vi "SaccadeAnalyser - Main.vi"(8 "error in (no error)":errorcluster, 11 "Data IN":T3={"Impulse Positions"=[{"Start"=5471, "End"=5813, "Impulse Plane"=enum."Yaw", "Impulse Direction +ve?"=FALSE, "Time offset"=0, "Amplitude offset"=0.0}, {"Start"=6974, "End"=7325, "Impulse Plane"=enum."Yaw", "Impulse Direction +ve?"=TRUE, "Time offset"=0, "Amplitude offset"=0.0}, {"Start"=7641, "End"=7980, "Impulse Plane"=enum."Yaw", "Impulse Direction +ve?"=FALSE, "Time offset"=0, "Amplitude offset"=0.0}, {"Start"=9060, "End"=9400, "Impulse Plane"=enum."Yaw", "Impulse Direction +ve?"=FALSE, "Time offset"=0, "Amplitude offset"=0.0}, {"Start"=9938, "End"=10282, "Impulse Plane"=enum."Yaw", "Impulse Direction +ve?"=FALSE, "Time offset"=0, "Amplitude offset"=0.0}, {"Start"=10800, "End"=11142, "Impulse Plane"=enum."Yaw", "Impulse Direction +ve?"=FALSE, "Time offset"=0, "Amplitude offset"=0.0}, {"Start"=11602, "End"=11942, "Impulse Plane"=enum."Yaw", "Impulse Direction +ve?"=TRUE, "Time offset"=0, "Amplitude offset"=0.0}, {"Start"=12449, "End"=12790, "Impulse Plane"=enum."Yaw", "Impulse Direction +ve?"=TRUE, "Time offset"=0, "Amplitude offset"=0.0}, {"Start"=13310, "End"=13653, "Impulse Plane"=enum."Yaw", "Impulse Direction +ve?"=TRUE, "Time offset"=0, "Amplitude offset"=0.0}, {"Start"=14191, "End"=14535, "Impulse Plane"=enum."Yaw", "Impulse Direction +ve?"=TRUE, "Time offset"=0, "Amplitude offset"=0.0}, {"Start"=15040, "End"=15380, "Impulse Plane"=enum."Yaw", "Impulse Direction +ve?"=FALSE, "Time offset"=0, "Amplitude offset"=0.0}, {"Start"=16780, "End"=17124, "Impulse Plane"=enum."Yaw", "Impulse Direction +ve?"=TRUE, "Time offset"=0, "Amplitude offset"=0.0}, {"Start"=17572, "End"=17913, "Impulse Plane"=enum."Yaw", "Impulse Direction +ve?"=FALSE, "Time offset"=0, "Amplitude offset"=0.0}, {"Start"=18369, "End"=18713, "Impulse Plane"=enum."Yaw", "Impulse Direction +ve?"=FALSE, "Time offset"=0, "Amplitude offset"=0.0}, {"Start"=19174, "End"=19519, "Impulse Plane"=enum."Yaw", "Impulse Direction +ve?"=FALSE, "Time offset"=0, "Amplitude offset"=0.0}, {"Start"=19928, "End"=20270, "Impulse Plane"=enum."Yaw", "Impulse Direction +ve?"=TRUE, "Time offset"=0, "Amplitude offset"=0.0}, {"Start"=20762, "End"=21121, "Impulse Plane"=enum."Yaw", "Impulse Direction +ve?"=FALSE, "Time offset"=0, "Amplitude offset"=0.0}, {"Start"=21554, "End"=21888, "Impulse Plane"=enum."Yaw", "Impulse Direction +ve?"=FALSE, "Time offset"=0, "Amplitude offset"=0.0}, {"Start"=22293, "End"=22639, "Impulse Plane"=enum."Yaw", "Impulse Direction +ve?"=TRUE, "Time offset"=0, "Amplitude offset"=0.0}, {"Start"=23109, "End"=23464, "Impulse Plane"=enum."Yaw", "Impulse Direction +ve?"=TRUE, "Time offset"=0, "Amplitude offset"=0.0}, {"Start"=23868, "End"=24215, "Impulse Plane"=enum."Yaw", "Impulse Direction +ve?"=TRUE, "Time offset"=0, "Amplitude offset"=0.0}, {"Start"=24643, "End"=24992, "Impulse Plane"=enum."Yaw", "Impulse Direction +ve?"=FALSE, "Time offset"=0, "Amplitude offset"=0.0}, {"Start"=25685, "End"=26023, "Impulse Plane"=enum."Yaw", "Impulse Direction +ve?"=FALSE, "Time offset"=0, "Amplitude offset"=0.0}, {"Start"=26431, "End"=26768, "Impulse Plane"=enum."Yaw", "Impulse Direction +ve?"=FALSE, "Time offset"=0, "Amplitude offset"=0.0}, {"Start"=27251, "End"=27595, "Impulse Plane"=enum."Yaw", "Impulse Direction +ve?"=FALSE, "Time offset"=0, "Amplitude offset"=0.0}, {"Start"=28832, "End"=29180, "Impulse Plane"=enum."Yaw", "Impulse Direction +ve?"=TRUE, "Time offset"=0, "Amplitude offset"=0.0}, {"Start"=31028, "End"=31383, "Impulse Plane"=enum."LARP", "Impulse Direction +ve?"=FALSE, "Time offset"=0, "Amplitude offset"=0.0}, {"Start"=32603, "End"=32936, "Impulse Plane"=enum."LARP", "Impulse Direction +ve?"=TRUE, "Time offset"=0, "Amplitude offset"=0.0}, {"Start"=33445, "End"=33779, "Impulse Plane"=enum."LARP", "Impulse Direction +ve?"=TRUE, "Time offset"=0, "Amplitude offset"=0.0}, {"Start"=34276, "End"=34629, "Impulse Plane"=enum."LARP", "Impulse Direction +ve?"=FALSE, "Time offset"=0, "Amplitude offset"=0.0}, {"Start"=35114, "End"=35460, "Impulse Plane"=enum."LARP", "Impulse Direction +ve?"=FALSE, "Time offset"=0, "Amplitude offset"=0.0}, {"Start"=35981, "End"=36324, "Impulse Plane"=enum."LARP", "Impulse Direction +ve?"=TRUE, "Time offset"=0, "Amplitude offset"=0.0}, {"Start"=36920, "End"=37249, "Impulse Plane"=enum."LARP", "Impulse Direction +ve?"=TRUE, "Time offset"=0, "Amplitude offset"=0.0}, {"Start"=37988, "End"=38322, "Impulse Plane"=enum."LARP", "Impulse Direction +ve?"=TRUE, "Time offset"=0, "Amplitude offset"=0.0}, {"Start"=38964, "End"=39324, "Impulse Plane"=enum."LARP", "Impulse Direction +ve?"=FALSE, "Time offset"=0, "Amplitude offset"=0.0}, {"Start"=39948, "End"=40284, "Impulse Plane"=enum."LARP", "Impulse Direction +ve?"=TRUE, "Time offset"=0, "Amplitude offset"=0.0}, {"Start"=40958, "End"=41293, "Impulse Plane"=enum."LARP", "Impulse Direction +ve?"=TRUE, "Time offset"=0, "Amplitude offset"=0.0}, {"Start"=41899, "End"=42229, "Impulse Plane"=enum."LARP", "Impulse Direction +ve?"=TRUE, "Time offset"=0, "Amplitude offset"=0.0}, {"Start"=42801, "End"=43154, "Impulse Plane"=enum."LARP", "Impulse Direction +ve?"=FALSE, "Time offset"=0, "Amplitude offset"=0.0}, {"Start"=43641, "End"=43980, "Impulse Plane"=enum."LARP", "Impulse Direction +ve?"=TRUE, "Time offset"=0, "Amplitude offset"=0.0}, {"Start"=44466, "End"=44821, "Impulse Plane"=enum."LARP", "Impulse Direction +ve?"=FALSE, "Time offset"=0, "Amplitude offset"=0.0}, {"Start"=45388, "End"=45722, "Impulse Plane"=enum."LARP", "Impulse Direction +ve?"=TRUE, "Time offset"=0, "Amplitude offset"=0.0}, {"Start"=46149, "End"=46510, "Impulse Plane"=enum."LARP", "Impulse Direction +ve?"=FALSE, "Time offset"=0, "Amplitude offset"=0.0}, {"Start"=47874, "End"=48206, "Impulse Plane"=enum."LARP", "Impulse Direction +ve?"=TRUE, "Time offset"=0, "Amplitude offset"=0.0}, {"Start"=50143, "End"=50479, "Impulse Plane"=enum."RALP", "Impulse Direction +ve?"=TRUE, "Time offset"=0, "Amplitude offset"=0.0}, {"Start"=50976, "End"=51310, "Impulse Plane"=enum."RALP", "Impulse Direction +ve?"=FALSE, "Time offset"=0, "Amplitude offset"=0.0}, {"Start"=51892, "End"=52226, "Impulse Plane"=enum."RALP", "Impulse Direction +ve?"=FALSE, "Time offset"=0, "Amplitude offset"=0.0}, {"Start"=52839, "End"=53171, "Impulse Plane"=enum."RALP", "Impulse Direction +ve?"=FALSE, "Time offset"=0, "Amplitude offset"=0.0}, {"Start"=53676, "End"=54012, "Impulse Plane"=enum."RALP", "Impulse Direction +ve?"=TRUE, "Time offset"=0, "Amplitude offset"=0.0}, {"Start"=54530, "End"=54877, "Impulse Plane"=enum."RALP", "Impulse Direction +ve?"=FALSE, "Time offset"=0, "Amplitude offset"=0.0}, {"Start"=55371, "End"=55711, "Impulse Plane"=enum."RALP", "Impulse Direction +ve?"=TRUE, "Time offset"=0, "Amplitude offset"=0.0}, {"Start"=56153, "End"=56482, "Impulse Plane"=enum."RALP", "Impulse Direction +ve?"=FALSE, "Time offset"=0, "Amplitude offset"=0.0}, {"Start"=57053, "End"=57390, "Impulse Plane"=enum."RALP", "Impulse Direction +ve?"=FALSE, "Time offset"=0, "Amplitude offset"=0.0}, {"Start"=57954, "End"=58292, "Impulse Plane"=enum."RALP", "Impulse Direction +ve?"=FALSE, "Time offset"=0, "Amplitude offset"=0.0}, {"Start"=58794, "End"=59130, "Impulse Plane"=enum."RALP", "Impulse Direction +ve?"=TRUE, "Time offset"=0, "Amplitude offset"=0.0}, {"Start"=59587, "End"=59931, "Impulse Plane"=enum."RALP", "Impulse Direction +ve?"=TRUE, "Time offset"=0, "Amplitude offset"=0.0}, {"Start"=60399, "End"=60744, "Impulse Plane"=enum."RALP", "Impulse Direction +ve?"=FALSE, "Time offset"=0, "Amplitude offset"=0.0}, {"Start"=61218, "End"=61559, "Impulse Plane"=enum."RALP", "Impulse Direction +ve?"=FALSE, "Time offset"=0, "Amplitude offset"=0.0}, {"Start"=62100, "End"=62442, "Impulse Plane"=enum."RALP", "Impulse Direction +ve?"=FALSE, "Time offset"=0, "Amplitude offset"=0.0}, {"Start"=62989, "End"=63322, "Impulse Plane"=enum."RALP", "Impulse Direction +ve?"=FALSE, "Time offset"=0, "Amplitude offset"=0.0}, {"Start"=63787, "End"=64136, "Impulse Plane"=enum."RALP", "Impulse Direction +ve?"=TRUE, "Time offset"=0, "Amplitude offset"=0.0}, {"Start"=64603, "End"=64953, "Impulse Plane"=enum."RALP", "Impulse Direction +ve?"=FALSE, "Time offset"=0, "Amplitude offset"=0.0}, {"Start"=65462, "End"=65795, "Impulse Plane"=enum."RALP", "Impulse Direction +ve?"=FALSE, "Time offset"=0, "Amplitude offset"=0.0}, {"Start"=66308, "End"=66645, "Impulse Plane"=enum."RALP", "Impulse Direction +ve?"=FALSE, "Time offset"=0, "Amplitude offset"=0.0}, {"Start"=67052, "End"=67402, "Impulse Plane"=enum."RALP", "Impulse Direction +ve?"=TRUE, "Time offset"=0, "Amplitude offset"=0.0}], "No. Imp"=15, "Parameter Time Series"=[{"time offset"=0.0, "Offset"=0.0, "Gain"=1.0, "inverse"=FALSE, "filter data"=FALSE, "dots"=FALSE, "interpolate"=FALSE, "List 1"=5, "Color Box"=6618880, "Boolean"=TRUE}, {"time offset"=0.0, "Offset"=0.0, "Gain"=1.0, "inverse"=FALSE, "filter data"=FALSE, "dots"=FALSE, "interpolate"=FALSE, "List 1"=6, "Color Box"=6618880, "Boolean"=FALSE}, {"time offset"=0.0, "Offset"=0.0, "Gain"=1.0, "inverse"=FALSE, "filter data"=FALSE, "dots"=FALSE, "interpolate"=FALSE, "List 1"=7, "Color Box"=6618880, "Boolean"=FALSE}, {"time offset"=0.0, "Offset"=0.0, "Gain"=1.0, "inverse"=FALSE, "filter data"=FALSE, "dots"=FALSE, "interpolate"=FALSE, "List 1"=13, "Color Box"=16777224, "Boolean"=TRUE}, {"time offset"=0.0, "Offset"=0.0, "Gain"=1.0, "inverse"=FALSE, "filter data"=FALSE, "dots"=FALSE, "interpolate"=FALSE, "List 1"=14, "Color Box"=16777224, "Boolean"=FALSE}, {"time offset"=0.0, "Offset"=0.0, "Gain"=1.0, "inverse"=FALSE, "filter data"=FALSE, "dots"=FALSE, "interpolate"=FALSE, "List 1"=15, "Color Box"=16777224, "Boolean"=FALSE}], "Parameter Impuls Series"=[{"Color"=6618880, "Visible"=TRUE, "Channel"=1, "Invert"=FALSE, "Desaccade"=FALSE, "Offset"=0.0, "Gain"=1.0}, {"Color"=6618880, "Visible"=FALSE, "Channel"=6, "Invert"=FALSE, "Desaccade"=FALSE, "Offset"=0.0, "Gain"=1.0}, {"Color"=6618880, "Visible"=FALSE, "Channel"=7, "Invert"=FALSE, "Desaccade"=FALSE, "Offset"=0.0, "Gain"=1.0}, {"Color"=16777224, "Visible"=TRUE, "Channel"=13, "Invert"=FALSE, "Desaccade"=FALSE, "Offset"=0.0, "Gain"=1.0}, {"Color"=16777224, "Visible"=FALSE, "Channel"=14, "Invert"=FALSE, "Desaccade"=FALSE, "Offset"=0.0, "Gain"=1.0}, {"Color"=16777224, "Visible"=FALSE, "Channel"=15, "Invert"=FALSE, "Desaccade"=FALSE, "Offset"=0.0, "Gain"=1.0}], "Experiment Parameters"={"Freq"=0.0, "Vel"=0, "Acc"=0, "Stimulus"="Head Impulse"}, "Autosort File"=refnum, "Data File"={"Data Channels"=array34x71049[2415666 elements], "Sample Rate"=500, "Channel List"=["Hz Position-in-Head", "Hz Velocity-in-Head", "Hy Position-in-Head", "Hy Velocity-in-Head", "Hx Position-in-Head", "Hx Velocity-in-Head", "Hl Velocity-in-Head", "Hr Velocity-in-Head", "Lx Position-in-Head", "Ly Position-in-Head", "Lz Position-in-Head", "Lx Velocity-in-Head", "Ly Velocity-in-Head", "Lz Velocity-in-Head", "Ll Velocity-in-Head", "Lr Velocity-in-Head", "Rx Position-in-Head", "Ry Position-in-Head", "Rz Position-in-Head", "Rx Velocity-in-Head", "Ry Velocity-in-Head", "Rz Velocity-in-Head", "Rl Velocity-in-Head", "Rr Velocity-in-Head", "Target on/off", "aux input 1", "aux input 2", " ", "", "", "", "Target Hor", "Target Ver", ""]}, "Experiment data path"=path "C:/Users/w.figtree/Desktop/Coils Data/3", "Image data path"=path "/Macintosh HD/Users/patrick/Studium/Diploma Thesis/Data Analysis", "LVS data path"=path "/Macintosh HD/Users/patrick/Studium/Diploma Thesis/Data Analysis", "Raw copy path"=path "/Macintosh HD/Users/patrick/Studium/Diploma Thesis/Data Analysis", "filename"="passive_lvs.lvs", "desaccading parameters"={"Tolerance"=3, "Acc Range"=7000.0, "Sample Rate"=500, "Impulse Plane 2"=enum."Yaw", "Impulse dir"=FALSE}, "Experiment Parameters 2"={"Subject"="SE Trial Short Term", "Strain"="", "Rotation plane"="", "Experimenter"=" ", "Trial"=0.0, "Time"=0.0}, "Excel"={"Excel._Application"=refnum, "Use Excel"=TRUE, "Worksheet SINE"=refnum, "Row SINE"=0, "Worksheet TRANS"=refnum, "Row TRANS"=0}, "Session Config File"=refnum, "Autosort Parameter Set"=4, "EMA Version"="EMA 2016a", "desacc "={"Threshold 1 [Acc]"=7000.0, "Threshold 2 [% of TH1]"=60, "tolerance"=3, "Search WD "=0.1, " always use TH2"=FALSE, "Range"=3.0, "Max time"=120.0, "Min time"=20.0, "Velocity Threshold"=150}, "Cycle Nr for Saccades"={"POS"=0, "NEG"=0}, "calibration name"="u_calibration_1_p00001s001_calib.mat", "Excel"=refnum} {"Parameter Time Series"."time offset" format="%.3f"; "Parameter Time Series"."Gain" format="%.1f"; "Parameter Time Series"."Offset" format="%.1f"; "Parameter Time Series"."List 1" items=["Motor-Pos", "Motor-Vel", "Lx Position-in-Head", "Ly Position-in-Head", "Lz Position-in-Head", "Lx Velocity-in-Head", "Ly Velocity-in-Head", "Lz Velocity-in-Head", "Ll Velocity-in-Head", "Lr Velocity-in-Head", "Lx Accel-in-Head", "Ly Accel-in-Head", "Lz Accel-in-Head", "Rx Position-in-Head", "Ry Position-in-Head", "Rz Position-in-Head", "Rx Velocity-in-Head", "Ry Velocity-in-Head", "Rz Velocity-in-Head", "Rl Velocity-in-Head", "Rr Velocity-in-Head", "Rx Accel-in-Head", "Ry Accel-in-Head", "Rz Accel-in-Head", "Global Trigger", "", "", ""]; "Parameter Impuls Series"."Gain" format="%.1f"; "Parameter Impuls Series"."Offset" format="%.1f"}) -> (0 "error out":errorcluster, 3 "Data OUT":T3={"Impulse Positions"=[{"Start"=5471, "End"=5813, "Impulse Plane"=enum."Yaw", "Impulse Direction +ve?"=FALSE, "Time offset"=0, "Amplitude offset"=0.0}, {"Start"=6974, "End"=7325, "Impulse Plane"=enum."Yaw", "Impulse Direction +ve?"=TRUE, "Time offset"=0, "Amplitude offset"=0.0}, {"Start"=7641, "End"=7980, "Impulse Plane"=enum."Yaw", "Impulse Direction +ve?"=FALSE, "Time offset"=0, "Amplitude offset"=0.0}, {"Start"=9060, "End"=9400, "Impulse Plane"=enum."Yaw", "Impulse Direction +ve?"=FALSE, "Time offset"=0, "Amplitude offset"=0.0}, {"Start"=9938, "End"=10282, "Impulse Plane"=enum."Yaw", "Impulse Direction +ve?"=FALSE, "Time offset"=0, "Amplitude offset"=0.0}, {"Start"=10800, "End"=11142, "Impulse Plane"=enum."Yaw", "Impulse Direction +ve?"=FALSE, "Time offset"=0, "Amplitude offset"=0.0}, {"Start"=11602, "End"=11942, "Impulse Plane"=enum."Yaw", "Impulse Direction +ve?"=TRUE, "Time offset"=0, "Amplitude offset"=0.0}, {"Start"=12449, "End"=12790, "Impulse Plane"=enum."Yaw", "Impulse Direction +ve?"=TRUE, "Time offset"=0, "Amplitude offset"=0.0}, {"Start"=13310, "End"=13653, "Impulse Plane"=enum."Yaw", "Impulse Direction +ve?"=TRUE, "Time offset"=0, "Amplitude offset"=0.0}, {"Start"=14191, "End"=14535, "Impulse Plane"=enum."Yaw", "Impulse Direction +ve?"=TRUE, "Time offset"=0, "Amplitude offset"=0.0}, {"Start"=15040, "End"=15380, "Impulse Plane"=enum."Yaw", "Impulse Direction +ve?"=FALSE, "Time offset"=0, "Amplitude offset"=0.0}, {"Start"=16780, "End"=17124, "Impulse Plane"=enum."Yaw", "Impulse Direction +ve?"=TRUE, "Time offset"=0, "Amplitude offset"=0.0}, {"Start"=17572, "End"=17913, "Impulse Plane"=enum."Yaw", "Impulse Direction +ve?"=FALSE, "Time offset"=0, "Amplitude offset"=0.0}, {"Start"=18369, "End"=18713, "Impulse Plane"=enum."Yaw", "Impulse Direction +ve?"=FALSE, "Time offset"=0, "Amplitude offset"=0.0}, {"Start"=19174, "End"=19519, "Impulse Plane"=enum."Yaw", "Impulse Direction +ve?"=FALSE, "Time offset"=0, "Amplitude offset"=0.0}, {"Start"=19928, "End"=20270, "Impulse Plane"=enum."Yaw", "Impulse Direction +ve?"=TRUE, "Time offset"=0, "Amplitude offset"=0.0}, {"Start"=20762, "End"=21121, "Impulse Plane"=enum."Yaw", "Impulse Direction +ve?"=FALSE, "Time offset"=0, "Amplitude offset"=0.0}, {"Start"=21554, "End"=21888, "Impulse Plane"=enum."Yaw", "Impulse Direction +ve?"=FALSE, "Time offset"=0, "Amplitude offset"=0.0}, {"Start"=22293, "End"=22639, "Impulse Plane"=enum."Yaw", "Impulse Direction +ve?"=TRUE, "Time offset"=0, "Amplitude offset"=0.0}, {"Start"=23109, "End"=23464, "Impulse Plane"=enum."Yaw", "Impulse Direction +ve?"=TRUE, "Time offset"=0, "Amplitude offset"=0.0}, {"Start"=23868, "End"=24215, "Impulse Plane"=enum."Yaw", "Impulse Direction +ve?"=TRUE, "Time offset"=0, "Amplitude offset"=0.0}, {"Start"=24643, "End"=24992, "Impulse Plane"=enum."Yaw", "Impulse Direction +ve?"=FALSE, "Time offset"=0, "Amplitude offset"=0.0}, {"Start"=25685, "End"=26023, "Impulse Plane"=enum."Yaw", "Impulse Direction +ve?"=FALSE, "Time offset"=0, "Amplitude offset"=0.0}, {"Start"=26431, "End"=26768, "Impulse Plane"=enum."Yaw", "Impulse Direction +ve?"=FALSE, "Time offset"=0, "Amplitude offset"=0.0}, {"Start"=27251, "End"=27595, "Impulse Plane"=enum."Yaw", "Impulse Direction +ve?"=FALSE, "Time offset"=0, "Amplitude offset"=0.0}, {"Start"=28832, "End"=29180, "Impulse Plane"=enum."Yaw", "Impulse Direction +ve?"=TRUE, "Time offset"=0, "Amplitude offset"=0.0}, {"Start"=31028, "End"=31383, "Impulse Plane"=enum."LARP", "Impulse Direction +ve?"=FALSE, "Time offset"=0, "Amplitude offset"=0.0}, {"Start"=32603, "End"=32936, "Impulse Plane"=enum."LARP", "Impulse Direction +ve?"=TRUE, "Time offset"=0, "Amplitude offset"=0.0}, {"Start"=33445, "End"=33779, "Impulse Plane"=enum."LARP", "Impulse Direction +ve?"=TRUE, "Time offset"=0, "Amplitude offset"=0.0}, {"Start"=34276, "End"=34629, "Impulse Plane"=enum."LARP", "Impulse Direction +ve?"=FALSE, "Time offset"=0, "Amplitude offset"=0.0}, {"Start"=35114, "End"=35460, "Impulse Plane"=enum."LARP", "Impulse Direction +ve?"=FALSE, "Time offset"=0, "Amplitude offset"=0.0}, {"Start"=35981, "End"=36324, "Impulse Plane"=enum."LARP", "Impulse Direction +ve?"=TRUE, "Time offset"=0, "Amplitude offset"=0.0}, {"Start"=36920, "End"=37249, "Impulse Plane"=enum."LARP", "Impulse Direction +ve?"=TRUE, "Time offset"=0, "Amplitude offset"=0.0}, {"Start"=37988, "End"=38322, "Impulse Plane"=enum."LARP", "Impulse Direction +ve?"=TRUE, "Time offset"=0, "Amplitude offset"=0.0}, {"Start"=38964, "End"=39324, "Impulse Plane"=enum."LARP", "Impulse Direction +ve?"=FALSE, "Time offset"=0, "Amplitude offset"=0.0}, {"Start"=39948, "End"=40284, "Impulse Plane"=enum."LARP", "Impulse Direction +ve?"=TRUE, "Time offset"=0, "Amplitude offset"=0.0}, {"Start"=40958, "End"=41293, "Impulse Plane"=enum."LARP", "Impulse Direction +ve?"=TRUE, "Time offset"=0, "Amplitude offset"=0.0}, {"Start"=41899, "End"=42229, "Impulse Plane"=enum."LARP", "Impulse Direction +ve?"=TRUE, "Time offset"=0, "Amplitude offset"=0.0}, {"Start"=42801, "End"=43154, "Impulse Plane"=enum."LARP", "Impulse Direction +ve?"=FALSE, "Time offset"=0, "Amplitude offset"=0.0}, {"Start"=43641, "End"=43980, "Impulse Plane"=enum."LARP", "Impulse Direction +ve?"=TRUE, "Time offset"=0, "Amplitude offset"=0.0}, {"Start"=44466, "End"=44821, "Impulse Plane"=enum."LARP", "Impulse Direction +ve?"=FALSE, "Time offset"=0, "Amplitude offset"=0.0}, {"Start"=45388, "End"=45722, "Impulse Plane"=enum."LARP", "Impulse Direction +ve?"=TRUE, "Time offset"=0, "Amplitude offset"=0.0}, {"Start"=46149, "End"=46510, "Impulse Plane"=enum."LARP", "Impulse Direction +ve?"=FALSE, "Time offset"=0, "Amplitude offset"=0.0}, {"Start"=47874, "End"=48206, "Impulse Plane"=enum."LARP", "Impulse Direction +ve?"=TRUE, "Time offset"=0, "Amplitude offset"=0.0}, {"Start"=50143, "End"=50479, "Impulse Plane"=enum."RALP", "Impulse Direction +ve?"=TRUE, "Time offset"=0, "Amplitude offset"=0.0}, {"Start"=50976, "End"=51310, "Impulse Plane"=enum."RALP", "Impulse Direction +ve?"=FALSE, "Time offset"=0, "Amplitude offset"=0.0}, {"Start"=51892, "End"=52226, "Impulse Plane"=enum."RALP", "Impulse Direction +ve?"=FALSE, "Time offset"=0, "Amplitude offset"=0.0}, {"Start"=52839, "End"=53171, "Impulse Plane"=enum."RALP", "Impulse Direction +ve?"=FALSE, "Time offset"=0, "Amplitude offset"=0.0}, {"Start"=53676, "End"=54012, "Impulse Plane"=enum."RALP", "Impulse Direction +ve?"=TRUE, "Time offset"=0, "Amplitude offset"=0.0}, {"Start"=54530, "End"=54877, "Impulse Plane"=enum."RALP", "Impulse Direction +ve?"=FALSE, "Time offset"=0, "Amplitude offset"=0.0}, {"Start"=55371, "End"=55711, "Impulse Plane"=enum."RALP", "Impulse Direction +ve?"=TRUE, "Time offset"=0, "Amplitude offset"=0.0}, {"Start" (continued)
24.01261904812929, 23.428908269352068, 22.770019063649308, 22.069631838895774, 21.342156639794716, 20.595825623349075, 19.82784564052124, 19.021253878068407, 18.164106126567248, 17.254669892990364, 16.29777196822669, 15.311916965804672, 14.321665191423946, 13.345319491254823, 12.400091096315116, 11.50297679721817, 10.665610723933703, 9.889576422547204, 9.172144968094683, 8.513824696280961, 7.910353133186064, 7.351127756489129, 6.8244091696694245, 6.320045209874815, 5.839834201686308, 5.401280196007361, 5.036629363424687, 4.790495353288961, 4.69727667858808, 4.774637598433885, 5.030961736572146, 5.442368650274481, 5.948362522690943, 6.479605818763797, 6.968216502985549, 7.35889702039092, 7.6286912816653345, 7.7865738860185605, 7.87024006232021, 7.942925400093573, 8.069791600667854, 8.293500554118122, 8.628097701430264, 9.064016956166405, 9.560847897637844, 10.053275017498667, 10.479382048439597, 10.79618308610415, 10.980785150974793, 11.031807809002775, 10.974439568714224, 10.85027685937862, 10.698931083451729, 10.544684874085853, 10.38972248423801, 10.222996358180055, 10.026989023211396, 9.779890727330592, 9.464283777201032, 9.075015771680539, 8.627839810984055, 8.158272171420684, 7.704972342026168, 7.300256178592089, 6.973798720186207, 6.74522851902298, 6.612376316977297, 6.550864987706879, 6.52556929393932, 6.502105707691413, 6.4492130482105186, 6.352143457887497, 6.217411113194651, 6.0600853406327255, 5.903325995448299, 5.771334565188951, 5.681034973578413, 5.646709144906293, 5.663672674591531, 5.70702100302696, 5.751131894304083, 5.760438900534005, 5.696691827551424, 5.541591244197238, 5.286571420847984, 4.9325496467762004, 4.501243912157196, 4.032665404177671, 3.5779355494598377, 3.1914964620330863, 2.927529456512798, 2.823335970726199, 2.887833068463011, 3.1095550288323306, 3.4580825698320465, 3.88083581822546, 4.316307387581903, 4.710963642362774, 5.018945876487839, 5.206872843742943, 5.267180894956013, 5.213635734248885, 5.067231367237529, 4.861319937765559, 4.635413218212038, 4.4218144017034255, 4.2562938485177755, 4.169566890182191, 4.171688327155885, 4.256068700565624, 4.409496310467918, 4.612569046091239, 4.836635527731177, 5.047411031065907, 5.218589004102354, 5.346523047142081, 5.438944068485455, 5.510740500889582, 5.58576405688371, 5.681536308168757, 5.794503522785154, 5.902157219346062, 5.977230030494396, 5.9848846662034685, 5.890547457467175, 5.682265669147694, 5.375801635279512, 5.0203732988709175, 4.69430499025112, 4.479580312679319, 4.446221928897202, 4.6366354757890775, 5.0499511213979975, 5.641562130025068, 6.3308668196871105, 7.019196163072959, 7.6089513336487276, 8.03369783491815, 8.268583669923292, 8.32791692790262, 8.27399124574497, 8.192347825911343]}, {[0.0, 2.0, 4.0, 6.0, 8.0, 10.0, 12.0, 14.0, 16.0, 18.000000000000004, 20.0, 22.0, 24.0, 26.000000000000004, 28.0, 30.0, 32.0, 34.0, 36.00000000000001, 38.0, 40.0, 42.0, 44.0, 46.0, 48.0, 50.0, 52.00000000000001, 54.0, 56.0, 58.0, 60.0, 62.0, 64.0, 66.0, 68.0, 70.0, 72.00000000000001, 74.0, 76.0, 78.0, 80.0, 82.0, 84.0, 86.0, 88.0, 90.0, 92.0, 94.0, 96.0, 98.0, 100.0, 102.00000000000001, 104.00000000000001, 106.0, 108.0, 110.0, 112.0, 114.0, 116.0, 118.00000000000001, 120.0, 122.0, 124.0, 126.0, 128.0, 130.0, 132.0, 134.0, 136.0, 138.0, 140.0, 142.00000000000003, 144.00000000000003, 146.0, 148.0, 150.0, 152.0, 154.0, 156.0, 158.0, 160.0, 162.0, 164.0, 166.0, 168.0, 170.0, 172.0, 174.00000000000003, 176.0, 178.0, 180.0, 182.0, 184.0, 186.0, 188.0, 190.0, 192.0, 194.0, 196.0, 198.0, 200.0, 202.0, 204.00000000000003, 206.00000000000003, 208.00000000000003, 210.0, 212.0, 214.0, 216.0, 218.0, 220.0, 222.0, 224.0, 226.0, 228.0, 230.0, 232.0, 234.0, 236.00000000000003, 238.00000000000003, 240.0, 242.0, 244.0, 246.0, 248.0, 250.0, 252.0, 254.0, 256.0, 258.0, 260.0, 262.0, 264.0, 266.0, 268.0, 270.0, 272.0, 274.0, 276.0, 278.0, 280.0, 282.0, 284.00000000000006, 286.00000000000006, 288.00000000000006, 290.0, 292.0, 294.0, 296.0, 298.0, 300.0, 302.0, 304.0, 306.0, 308.0, 310.0, 312.0, 314.0, 316.0, 318.0, 320.0, 322.0, 324.0, 326.0, 328.0, 330.0, 332.0, 334.0, 336.0, 338.0, 340.0, 342.0, 344.0, 346.00000000000006, 348.00000000000006, 350.00000000000006, 352.0, 354.0, 356.0, 358.0, 360.0, 362.0, 364.0, 366.0, 368.0, 370.0, 372.0, 374.0, 376.0, 378.0, 380.0, 382.0, 384.0, 386.0, 388.0, 390.0, 392.0, 394.0, 396.0, 398.0, 400.0, 402.0, 404.0, 406.0, 408.00000000000006, 410.00000000000006, 412.00000000000006, 414.00000000000006, 416.00000000000006, 418.0, 420.0, 422.0, 424.0, 426.0, 428.0, 430.0, 432.0, 434.0, 436.0, 438.0, 440.0, 442.0, 444.0, 446.0, 448.0, 450.0, 452.0, 454.0, 456.0, 458.0, 460.0, 462.0, 464.0, 466.0, 468.0, 470.00000000000006, 472.00000000000006, 474.00000000000006, 476.00000000000006, 478.00000000000006, 480.0, 482.0, 484.0, 486.0, 488.0, 490.0, 492.0, 494.0, 496.0, 498.0, 500.0, 502.0, 504.0, 506.0, 508.0, 510.0, 512.0, 514.0, 516.0, 518.0, 520.0, 522.0, 524.0, 526.0, 528.0, 530.0, 532.0, 534.0, 536.0, 538.0, 540.0, 542.0, 544.0, 546.0, 548.0, 550.0, 552.0, 554.0, 556.0, 558.0, 560.0, 562.0, 564.0, 566.0000000000001, 568.0000000000001, 570.0000000000001, 572.0000000000001, 574.0000000000001, 576.0000000000001, 578.0, 580.0, 582.0, 584.0, 586.0, 588.0, 590.0, 592.0, 594.0, 596.0, 598.0, 600.0, 602.0, 604.0, 606.0, 608.0, 610.0, 612.0, 614.0, 616.0, 618.0, 620.0, 622.0, 624.0, 626.0, 628.0, 630.0, 632.0, 634.0, 636.0, 638.0, 640.0, 642.0, 644.0, 646.0, 648.0, 650.0, 652.0, 654.0, 656.0, 658.0, 660.0, 662.0, 664.0, 666.0, 668.0], [-0.10553120933570703, -0.08400333126697923, -0.06084521968970513, -0.037506879812259086, -0.005225519412065616, 0.04482456389572409, 0.12470447179164168, 0.23966117888181948, 0.3687158800694075, 0.4775541016515792, 0.5246319102526256, 0.460040923309057, 0.23884543381811696, -0.1586143094681649, -0.7163042007305549, -1.3787379158841322, -2.0517450846309124, -2.6186210739206626, -2.9617713910987202, -2.9958394247591276, -2.697515941641182, -2.1244885211076276, -1.4096582510659061, -0.7306569469370885, -0.2738482069982169, -0.19187290468091867, -0.5582829907052105, -1.3315568280752537, -2.357900245473459, -3.4103591273092757, -4.245197598892631, -4.659789670853373, -4.5453539081611325, -3.920282167135543, -2.9262664208154003, -1.7909006148173106, -0.7642332351058041, -0.05751949075316887, 0.20877877155691138, 0.04152428141888542, -0.43823451752211895, -1.03919812874015, -1.5516742087844015, -1.8121703114108119, -1.7497446311852123, -1.3907475598931516, -0.8517093031193284, -0.30673212822438956, 0.0769957344956742, 0.18426450077038403, -0.017542432567125843, -0.4655582013710866, -1.0319033173462646, -1.5644506232635917, -1.9283447158799536, -2.045172190793343, -1.9000733871819193, -1.5406873425081598, -1.0603410864880916, -0.5579721730184035, -0.11412008795757878, 0.233760511021889, 0.5004320530885797, 0.7328640084282623, 0.9907971433206435, 1.330232702616184, 1.790627705138916, 2.382348313268446, 3.090355969154532, 3.89149028796944, 4.766263109572754, 5.698597408674404, 6.683455271084595, 7.742229238932255, 8.907954581699617, 10.209373559727506, 11.680557030411967, 13.3559521466179, 15.268411067988158, 17.453851696787584, 19.94275470602321, 22.769708895472093, 25.97205389119289, 29.57432608769504, 33.58407880808603, 37.99858201679099, 42.8083703874524, 47.98395597529881, 53.48495032152595, 59.280826356538654, 65.3421034141801, 71.63545040671113, 78.12569000239381, 84.75777704602545, 91.44282303954367, 98.07412044610243, 104.5417135830397, 110.73303748040857, 116.55846906150347, 121.9742718976011, 126.98722106727712, 131.64087046011576, 135.98673138461885, 140.06788317521955, 143.88504541576123, 147.38497293239854, 150.4824542128305, 153.0656035074012, 155.03347444982813, 156.34461376258457, 157.0153981911935, 157.11868487268964, 156.7853132951468, 156.15713453311452, 155.33060793455508, 154.3332614317673, 153.12366261012147, 151.59541089471983, 149.6002538589897, 147.00139882217002, 143.7279459866911, 139.8036245748391, 135.3369313984742, 130.5096703433158, 125.54098078600231, 120.61610806142733, 115.85220683588759, 111.27650463583535, 106.81591083301244, 102.33052273335018, 97.6666537298168, 92.70336885080819, 87.38062112451811, 81.7159629255708, 75.80122636475947, 69.77992895949589, 63.80980979165295, 58.02233723072696, 52.50621822876454, 47.30430923440218, 42.410413291113755, 37.78325799275856, 33.372319520111525, 29.13580655564173, 25.05260468516136, 21.124571576801348, 17.369554080506266, 13.820937189340045, 10.51450986280934, 7.471570782648957, 4.711755590173021, 2.2426313198102923, 0.039645895336986925, -1.9303157432340061, -3.7032662670090177, -5.327461310977329, -6.844143715641225, -8.286429115605365, -9.682005147415868, -11.027455895820776, -12.29845733175419, -13.470283405854557, -14.50391809687549, -15.350749000654417, -15.97665773706939, -16.371061206570893, -16.54125593775632, -16.50646890154465, -16.29787664913959, -15.956833060323266, -15.52614079397309, -15.038222630549319, -14.519858233257578, -13.995514105568276, -13.470072676696946, -12.936652646700336, -12.383095375057218, -11.783390637907507, -11.115069687962533, -10.3658816141141, -9.522409304861066, -8.589590748533677, -7.608928249506862, -6.639856775769532, -5.742354350596807, -4.972111303879556, -4.368330005595926, -3.941581129764627, -3.6696315244346476, -3.5019357394197215, -3.3816388551672656, -3.265669025611162, -3.135304122410094, -3.006642256124291, -2.925442039500874, -2.944473292754372, -3.1116913293418555, -3.443414885324179, -3.9054383740756276, -4.429838114553337, -4.9183022237033365, -5.273345073277001, -5.4460140322751105, -5.430088592320409, -5.259256417392174, -5.0251640568373475, -4.839917907760246, -4.7881551421286135, -4.924857444590882, -5.255349373882261, -5.723656543952083, -6.242108304695993, -6.719457157996956, -7.088404564952985, -7.319606400769368, -7.4256298070695905, -7.459881786332922, -7.489844901297074, -7.567655285082369, -7.709997011011911, -7.8901725728643815, -8.040749594057953, -8.066844094813941, -7.881611175536853, -7.432025913741137, -6.713286811368302, -5.780401332158699, -4.737028336491937, -3.713975595786512, -2.8410692483637243, -2.2086763410385997, -1.8535263425918842, -1.7625366514098342, -1.8709831534722907, -2.081883904121626, -2.2920269460635305, -2.4057090794371794, -2.352159661773735, -2.090296056670035, -1.6046650639716438, -0.9084204915576854, -0.041345593422326354, 0.931620863542554, 1.907975279501325, 2.7423150036557304, 3.2683343970762917, 3.3199922098449814, 2.7717317808631847, 1.610078145325277, -0.012091313230288447, -1.7421638804518995, -3.0389623640143157, -3.245396673757427, -1.6948480326152768, 2.1384328191819306, 8.469521915823595, 17.087054841087145, 27.315418397717107, 38.05757322742741, 47.94620610349132, 55.57948276025742, 59.777197966332054, 59.80311209652382, 55.50908234625477, 47.38023657915541, 36.450375305358186, 24.101455072542254, 11.809603266892601, 0.8926245665691606, -7.699270570892281, -13.502462377823814, -16.541721280039642, -17.24392262332151, -16.284433481949875, -14.412508844326226, -12.2971280291156, -10.413033131950677, -8.996578679830302, -8.065908034032386, -7.492233682316934, -7.083877872231896, -6.659918661478668, -6.108617823230636, -5.409952212505134, -4.6257609802418695, -3.8702451865477783, -3.269539380732014, -2.918895706244002, -2.8533713477361964, -3.036998400644217, -3.375959011320643, -3.744399053256826, -4.007361386470827, -4.058913867283884, -3.8477029077907265, -3.381613811752663, -2.732053487618276, -2.0188574522191702, -1.3808772755247805, -0.9470251479473497, -0.8078555017105491, -0.9971620595453038, -1.4835945923590836, -2.1798741260680723, -2.9661199055637657, -3.7121268430453926, -4.30646398208801, -4.6797518451560425, -4.817394591663838, -4.753197166979762, -4.5549705865735515, -4.307418270038013, -4.086721346765543, -3.9475996897781958, -3.9103018580453455, -3.9628431746388175, -4.0795051098652655, -4.2298343073036655, -4.38647747861612, -4.537430882985264, -4.690725941790954, -4.857120270155013, -5.04866557419951, -5.275232107005449, -5.529637250815332, -5.797613971026762, -6.05583102763301, -6.27229204257479, -6.420744961737212, -6.492969917498198, -6.491518056898129, -6.416071883889407, -6.273291510227602, -6.074242310114257]}, {[0.0, 2.0, 4.0, 6.0, 8.0, 10.0, 12.0, 14.0, 16.0, 18.000000000000004, 20.0, 22.0, 24.0, 26.000000000000004, 28.0, 30.0, 32.0, 34.0, 36.00000000000001, 38.0, 40.0, 42.0, 44.0, 46.0, 48.0, 50.0, 52.00000000000001, 54.0, 56.0, 58.0, 60.0, 62.0, 64.0, 66.0, 68.0, 70.0, 72.00000000000001, 74.0, 76.0, 78.0, 80.0, 82.0, 84.0, 86.0, 88.0, 90.0, 92.0, 94.0, 96.0, 98.0, 100.0, 102.00000000000001, 104.00000000000001, 106.0, 108.0, 110.0, 112.0, 114.0, 116.0, 118.00000000000001, 120.0, 122.0, 124.0, 126.0, 128.0, 130.0, 132.0, 134.0, 136.0, 138.0, 140.0, 142.00000000000003, 144.00000000000003, 146.0, 148.0, 150.0, 152.0, 154.0, 156.0, 158.0, 160.0, 162.0, 164.0, 166.0, 168.0, 170.0, 172.0, 174.00000000000003, 176.0, 178.0, 180.0, 182.0, 184.0, 186.0, 188.0, 190.0, 192.0, 194.0, 196.0, 198.0, 200.0, 202.0, 204.00000000000003, 206.00000000000003, 208.00000000000003, 210.0, 212.0, 214.0, 216.0, 218.0, 220.0, 222.0, 224.0, 226.0, 228.0, 230.0, 232.0, 234.0, 236.00000000000003, 238.00000000000003, 240.0, 242.0, 244.0, 246.0, 248.0, 250.0, 252.0, 254.0, 256.0, 258.0, 260.0, 262.0, 264.0, 266.0, 268.0, 270.0, 272.0, 274.0, 276.0, 278.0, 280.0, 282.0, 284.00000000000006, 286.00000000000006, 288.00000000000006, 290.0, 292.0, 294.0, 296.0, 298.0, 300.0, 302.0, 304.0, 306.0, 308.0, 310.0, 312.0, 314.0, 316.0, 318.0, 320.0, 322.0, 324.0, 326.0, 328.0, 330.0, 332.0, 334.0, 336.0, 338.0, 340.0, 342.0, 344.0, 346.00000000000006, 348.00000000000006, 350.00000000000006, 352.0, 354.0, 356.0, 358.0, 360.0, 362.0, 364.0, 366.0, 368.0, 370.0, 372.0, 374.0, 376.0, 378.0, 380.0, 382.0, 384.0, 386.0, 388.0, 390.0, 392.0, 394.0, 396.0, 398.0, 400.0, 402.0, 404.0, 406.0, 408.00000000000006, 410.00000000000006, 412.00000000000006, 414.00000000000006, 416.00000000000006, 418.0, 420.0, 422.0, 424.0, 426.0, 428.0, 430.0, 432.0, 434.0, 436.0, 438.0, 440.0, 442.0, 444.0, 446.0, 448.0, 450.0, 452.0, 454.0, 456.0, 458.0, 460.0, 462.0, 464.0, 466.0, 468.0, 470.00000000000006, 472.00000000000006, 474.00000000000006, 476.00000000000006, 478.00000000000006, 480.0, 482.0, 484.0, 486.0, 488.0, 490.0, 492.0, 494.0, 496.0, 498.0, 500.0, 502.0, 504.0, 506.0, 508.0, 510.0, 512.0, 514.0, 516.0, 518.0, 520.0, 522.0, 524.0, 526.0, 528.0, 530.0, 532.0, 534.0, 536.0, 538.0, 540.0, 542.0, 544.0, 546.0, 548.0, 550.0, 552.0, 554.0, 556.0, 558.0, 560.0, 562.0, 564.0, 566.0000000000001, 568.0000000000001, 570.0000000000001, 572.0000000000001, 574.0000000000001, 576.0000000000001, 578.0, 580.0, 582.0, 584.0, 586.0, 588.0, 590.0, 592.0, 594.0, 596.0, 598.0, 600.0, 602.0, 604.0, 606.0, 608.0, 610.0, 612.0, 614.0, 616.0, 618.0, 620.0, 622.0, 624.0, 626.0, 628.0, 630.0, 632.0, 634.0, 636.0, 638.0, 640.0, 642.0, 644.0, 646.0, 648.0, 650.0, 652.0, 654.0, 656.0, 658.0, 660.0, 662.0, 664.0, 666.0, 668.0], [0.007518886437217098, -0.001524926879841626, -0.011825684121857805, -0.016901102805852553, -0.015516121026260876, -0.008712869725938432, 0.001647416785009348, 0.011409026447601889, 0.018935233259700368, 0.021188943156988493, 0.01379484842364942, -0.004311304724745391, -0.026268870558055823, -0.04262199870436412, -0.04552197729852736, -0.028998555263990866, 0.0052195960843750555, 0.04756255301784407, 0.081102548312602, 0.09381075381161885, 0.0865952350684065, 0.07705952580238762, 0.1002705096639005, 0.19606139053401606, 0.3971917424335256, 0.7199328348469756, 1.150482740021186, 1.63075072865022, 2.0702269818962096, 2.370951658586268, 2.4502977818130454, 2.2654426545245743, 1.829072921327601, 1.2107518921859013, 0.5224557174165048, -0.10846391862045568, -0.5716542714288773, -0.799539625281263, -0.7864961347032016, -0.5939909342358978, -0.3285241183129721, -0.11075922722705323, -0.04481412141960828, -0.18871851598777178, -0.5350763946557984, -1.014375952631521, -1.5154749260338525, -1.9130408693643368, -2.105438842939136, -2.039940449417623, -1.7285960096185677, -1.2528375585295493, -0.731028058110291, -0.28782835071261337, -0.028963550557271844, -0.008636568470422379, -0.22786163512712543, -0.6389515158617725, -1.1540957072082998, -1.6771045217479674, -2.1302006170468077, -2.4715643911908227, -2.6981561043681657, -2.8418365034342123, -2.9583487892956546, -3.1120988237225147, -3.3647442323275625, -3.7604050885871247, -4.3237518919123525, -5.05999678781134, -5.958411958938099, -6.994734947015251, -8.136666392417041, -9.364146700810185, -10.667836375132115, -12.04001475588461, -13.487904275921016, -15.04086439961403, -16.7458089940566, -18.66680401138332, -20.882645730664866, -23.48081450528266, -26.546616970160432, -30.148381642510884, -34.32159636926133, -39.06447449879012, -44.33295305475547, -50.037003497953414, -56.060863359835935, -62.28344742055911, -68.58900180182037, -74.87968519467736, -81.08228713418376, -87.14350276120032, -93.01766994101226, -98.66460841997349, -104.04800823383914, -109.12416903911051, -113.85328726064594, -118.20718143116076, -122.16812409957276, -125.72809505120091, -128.87722740218285, -131.6051633059846, -133.88624735358943, -135.67873573385194, -136.9479463390219, -137.6643388513372, -137.82040073196552, -137.44996457671277, -136.62422537421068, -135.44770649159537, -134.04465332641547, -132.53013640103944, -130.9762299069521, -129.40061829544769, -127.76993584985667, -126.00250278512944, -123.98609194732924, -121.61287110405951, -118.8170115854592, -115.58983455083013, -111.97298717793892, -108.05714668818898, -103.96278955243056, -99.79123023862093, -95.60277494400754, -91.41363129333638, -87.18823503295778, -82.85219734836002, -78.32716708517282, -73.55827759689578, -68.53257868928644, -63.29159810958005, -57.92371610483936, -52.551419875022766, -47.3051965296992, -42.295708918915885, -37.60260272823966, -33.26298677856039, -29.271764924247243, -25.5934633017075, -22.173809004646223, -18.953786678316064, -15.880100794423297, -12.914501113411204, -10.031299693428894, -7.213821522564435, -4.458925563398538, -1.7738147274165812, 0.8173644482901026, 3.2754917540012944, 5.556662545269458, 7.607545743639629, 9.37596008684572, 10.825204798083135, 11.936799906043861, 12.720166917498581, 13.214756858410816, 13.476573323429538, 13.568973022553113, 13.554057223383762, 13.476858619531658, 13.357400683789262, 13.19877069083228, 12.99059633455305, 12.709307990258512, 12.329571047012749, 11.8386373742722, 11.244291584759427, 10.566459227956754, 9.830711967171919, 9.07157012660388, 8.321758739374948, 7.593920455194107, 6.887983107723301, 6.196961039294319, 5.500109505172105, 4.779909624706402, 4.033943614930886, 3.2695456534649026, 2.5116096418157774, 1.8036692646927133, 1.1919100081380343, 0.7115779647790479, 0.37752012514703637, 0.18114419099074652, 0.09219739138283067, 0.06302691149179118, 0.04720058437952801, 0.02140861261185556, -0.010323432189998982, -0.0142344532229437, 0.06876937632892322, 0.30115892703499725, 0.721614934954971, 1.3322656936552608, 2.08563585790246, 2.880933283729332, 3.593109830142801, 4.094505695217565, 4.289509047092002, 4.158697481641173, 3.7530091965548804, 3.1736573984648597, 2.5680671450345445, 2.090116702736932, 1.8488218871337176, 1.8947185685809345, 2.2118433700016205, 2.723141378263988, 3.3200743227344756, 3.894251413777363, 4.365942324076688, 4.700584305950853, 4.909381344932921, 5.037369632049126, 5.1398180402174205, 5.257430376123928, 5.402523918261627, 5.553734540339276, 5.661819093434138, 5.667841341455255, 5.526220506796059, 5.216732795555363, 4.746695517377809, 4.151854425573735, 3.489800428741651, 2.827022984718157, 2.218923142199267, 1.6979816365252909, 1.2782226481160877, 0.9609840561343055, 0.7397610775962764, 0.6034514407159637, 0.5362570815602573, 0.517992397130127, 0.5214479765641813, 0.5042964674965659, 0.4136154531133579, 0.20131670075305208, -0.16807079109219386, -0.7064380134167371, -1.3874329119129558, -2.1450206022912908, 